vi "TLB Native Dynamic Events ver 0.26e.vi"() -> ()   [LabVIEW 2018] (continued)
                # "Stays in Task 5D until the object is detected"
                # "T: Go back to idle, F: Continue with task\""
                # ">> Manual override >>"
                n445 = case shown="False" w1151 {
                  tunnel: [w1164 w1170] -> w1160
                  tunnel: w1152 -> [w1162 w1168]
                  frame False {
                    n446 = for {
                      tunnel: string[] ["START TIMER", "OPEN CLAW", ""] ("element") -> [w1165] mode=indexing
                      shift-right: [w1167] -> w1164
                      shift-left: w1162 -> [w1166]
                      n447 = Enqueue Element(queue=w1166, element=w1165) -> (queue out=w1167:refnum<queue>)  [unwired: 2 in, 2 out]
                    }
                  }
                  frame True {
                    n448 = for {
                      shift-right: [w1172] -> w1170
                      shift-left: w1168 -> [w1173]
                      tunnel: string[] ["CAM CLOSE", "", ""] -> [w1171] mode=indexing
                      n449 = Enqueue Element(queue=w1173, element=w1171) -> (queue out=w1172:refnum<queue>)  [unwired: 2 in, 2 out]
                    }
                  }
                }
                n450 = Or(x=w1151, y=w1156) -> (x .or. y?=w1158:bool)
                n451 = Select(t=State_Type_Definitions,_for_0.26g_versions_and_later_2."True Stop" ("Enum"), s=w1156, f=State_Type_Definitions,_for_0.26g_versions_and_later_2."True Stop" ("Enum")) -> (s? t:f=w1153:T18)
                n452 = Select(t=w1153, s=w1158, f=State_Type_Definitions,_for_0.26g_versions_and_later_2."Task 5D" ("Enum")) -> (s? t:f=w1157:T18)
              }
              frame "Exit" {
                n453 = for {
                  shift-right: [w1180] -> w1177
                  shift-left: w1174 -> [w1181]
                  tunnel: string[] ["STOP", "RESET ENCODERS", "RESET YAW", "ARDUINO MODE 0"] -> [w1179] mode=indexing
                  n454 = Enqueue Element(queue=w1181, element=w1179) -> (queue out=w1180:refnum<queue>)  [unwired: 2 in, 2 out]
                }
              }
            }
          }
          frame 20 {
            # ">>> yStepper command>>>"
            n455 = Dequeue Element(queue=w1195, timeout in ms (-1)=w1196, error in (no error)=w1197) -> (element=w1199:T10)  [unwired: 3 out]
            n456 = formula code="if (pos < 100)\ny = 41;\n\nelse if (pos >= 100 && pos <= 140)\ny = 30;\n\nelse if (pos >= 141 && pos <= 170)\ny = 25;\n\nelse if (pos >= 171 &&pos <= 180) \ny = 20;\n\nelse if (pos >= 181&& pos <= 200)\ny = 15;\n\nelse if (pos >= 201 && pos <= 230)\ny = 10;\n\nelse if (pos >= 231 && pos <= 320)\ny = 8;\n\nelse if (pos > 320)\ny = 0;"("pos"=w1187) -> ("y"=w1190:dbl)
            n457 = To Unsigned Byte Integer(number=w1190) -> (unsigned 8bit integer=w1185:u8)
            n458 = Equal?(x=w1186, y=w1185) -> (x = y?=w1184:bool)
            n459 = case shown="\"Start Task 1\", Default" w1199 {
              tunnel: [w1206 State_Type_Definitions,_for_0.26g_versions_and_later_2."True Stop" ("Enum")] -> w1193
              tunnel: [w1209 w1226] -> w1191
              tunnel: [State_Type_Definitions,_for_0.26g_versions_and_later_2."Idle" ("Enum") State_Type_Definitions,_for_0.26g_versions_and_later_2."Shutdown" ("Enum")] -> w1192
              tunnel: w1198 -> [w1205 _]
              tunnel: w1194 -> [w1201 w1223]
              tunnel: w1184 -> [w1200 _]
              frame "Start Task 1", Default {
                # ">> T: Breaks out of state loop; F: Stays in loop>>"
                # ">> Manual override >>"
                # ">> Checks if time is up>>"
                # "Stays in Task 5D until the object is detected"
                # "T: Go back to idle, F: Continue with task\""
                # ">> Manual override >>"
                n460 = case shown="False" w1200 {
                  tunnel: [w1213 w1219] -> w1209
                  tunnel: w1201 -> [w1211 w1217]
                  frame False {
                    n461 = for {
                      tunnel: string[] ["READ STEPPER VALUES", "Y STEPPER CONTROL", ""] ("element") -> [w1214] mode=indexing
                      shift-right: [w1216] -> w1213
                      shift-left: w1211 -> [w1215]
                      n462 = Enqueue Element(queue=w1215, element=w1214) -> (queue out=w1216:refnum<queue>)  [unwired: 2 in, 2 out]
                    }
                  }
                  frame True {
                    n463 = for {
                      shift-right: [w1221] -> w1219
                      shift-left: w1217 -> [w1222]
                      tunnel: string[] ["CAM CLOSE", "DISPOSE BUFFERS", ""] -> [w1220] mode=indexing
                      n464 = Enqueue Element(queue=w1222, element=w1220) -> (queue out=w1221:refnum<queue>)  [unwired: 2 in, 2 out]
                    }
                  }
                }
                n465 = Or(x=w1200, y=w1205) -> (x .or. y?=w1207:bool)
                n466 = Select(t=State_Type_Definitions,_for_0.26g_versions_and_later_2."True Stop" ("Enum"), s=w1205, f=State_Type_Definitions,_for_0.26g_versions_and_later_2."Task 5F: ARM GRAB HEIGHT" ("Enum")) -> (s? t:f=w1202:T18)
                n467 = Select(t=w1202, s=w1207, f=State_Type_Definitions,_for_0.26g_versions_and_later_2."Task 5E: POSITION ARM" ("Enum")) -> (s? t:f=w1206:T18)
              }
              frame "Exit" {
                n468 = for {
                  shift-right: [w1229] -> w1226
                  shift-left: w1223 -> [w1230]
                  tunnel: string[] ["STOP", "RESET ENCODERS", "RESET YAW", "ARDUINO MODE 0"] -> [w1228] mode=indexing
                  n469 = Enqueue Element(queue=w1230, element=w1228) -> (queue out=w1229:refnum<queue>)  [unwired: 2 in, 2 out]
                }
              }
            }
            n470 = Bundle By Name(cluster=w1189, "yStepper desired"=w1185) -> (w1188:T20)
          }
          frame 21 {
            # ">>> Motor control cluster >>>"
            # ">>> yStepper command>>>"
            # ">> Manual override >>"
            n471 = Dequeue Element(queue=w1241, timeout in ms (-1)=w1240, error in (no error)=w1242) -> (element=w1239:T10)  [unwired: 3 out]
            n472 = Equal?(x=w1238, y=u8 1) -> (x = y?=w1236:bool)
            n473 = case shown="\"Start Task 1\", Default" w1239 {
              tunnel: [w1252 State_Type_Definitions,_for_0.26g_versions_and_later_2."True Stop" ("Enum")] -> w1243
              tunnel: [w1255 w1272] -> w1244
              tunnel: [State_Type_Definitions,_for_0.26g_versions_and_later_2."Idle" ("Enum") State_Type_Definitions,_for_0.26g_versions_and_later_2."Shutdown" ("Enum")] -> w1245
              tunnel: w1236 -> [w1251 _]
              tunnel: w1235 -> [w1250 _]
              tunnel: w1234 -> [w1246 w1269]
              frame "Start Task 1", Default {
                # "Stays in Task 5F until stepper reaches desired \nheight"
                # "T: Go back to idle, F: Continue with task\""
                # ">> Manual override >>"
                n474 = case shown="True" w1251 {
                  tunnel: [w1259 w1265] -> w1255
                  tunnel: w1246 -> [w1257 w1263]
                  frame False {
                    n475 = for {
                      tunnel: string[] ["Z STEPPER GRAB HEIGHT", "READ STEPPER VALUES"] ("element") -> [w1260] mode=indexing
                      shift-right: [w1262] -> w1259
                      shift-left: w1257 -> [w1261]
                      n476 = Enqueue Element(queue=w1261, element=w1260) -> (queue out=w1262:refnum<queue>)  [unwired: 2 in, 2 out]
                    }
                  }
                  frame True {
                    n477 = for {
                      shift-right: [w1267] -> w1265
                      shift-left: w1263 -> [w1268]
                      tunnel: string[] ["SET TIMER 5", "CLOSE CLAW", ""] -> [w1266] mode=indexing
                      n478 = Enqueue Element(queue=w1268, element=w1266) -> (queue out=w1267:refnum<queue>)  [unwired: 2 in, 2 out]
                    }
                  }
                }
                n479 = Or(x=w1251, y=w1250) -> (x .or. y?=w1253:bool)
                n480 = Select(t=State_Type_Definitions,_for_0.26g_versions_and_later_2."True Stop" ("Enum"), s=w1250, f=State_Type_Definitions,_for_0.26g_versions_and_later_2."Task 5G: CLOSE CLAW" ("Enum")) -> (s? t:f=w1247:T18)
                n481 = Select(t=w1247, s=w1253, f=State_Type_Definitions,_for_0.26g_versions_and_later_2."Task 5F: ARM GRAB HEIGHT" ("Enum")) -> (s? t:f=w1252:T18)
              }
              frame "Exit" {
                n482 = for {
                  shift-right: [w1275] -> w1272
                  shift-left: w1269 -> [w1276]
                  tunnel: string[] ["STOP", "RESET ENCODERS", "RESET YAW", "ARDUINO MODE 0"] -> [w1274] mode=indexing
                  n483 = Enqueue Element(queue=w1276, element=w1274) -> (queue out=w1275:refnum<queue>)  [unwired: 2 in, 2 out]
                }
              }
            }
          }
          frame 22 {
            # ">>> yStepper command>>>"
            # ">> Manual override >>"
            n484 = Dequeue Element(queue=w1287, timeout in ms (-1)=w1286, error in (no error)=w1285) -> (element=w1284:T10)  [unwired: 3 out]
            n485 = case shown="\"Start Task 1\", Default" w1284 {
              tunnel: [w1296 State_Type_Definitions,_for_0.26g_versions_and_later_2."True Stop" ("Enum")] -> w1289
              tunnel: [w1299 w1316] -> w1282
              tunnel: [State_Type_Definitions,_for_0.26g_versions_and_later_2."Idle" ("Enum") State_Type_Definitions,_for_0.26g_versions_and_later_2."Shutdown" ("Enum")] -> w1281
              tunnel: w1283 -> [w1290 _]
              tunnel: w1288 -> [w1295 w1313]
              tunnel: w1279 -> [w1294 _]
              frame "Start Task 1", Default {
                # ">> Is time up? >>"
                # "Determines if object is in range to pick up"
                # ">> Manual override >>"
                n486 = case shown="True" w1294 {
                  tunnel: [w1303 w1309] -> w1299
                  tunnel: w1295 -> [w1301 w1307]
                  frame False {
                    n487 = for {
                      tunnel: string[] ["CLOSE CLAW", "START TIMER"] ("element") -> [w1304] mode=indexing
                      shift-right: [w1306] -> w1303
                      shift-left: w1301 -> [w1305]
                      n488 = Enqueue Element(queue=w1305, element=w1304) -> (queue out=w1306:refnum<queue>)  [unwired: 2 in, 2 out]
                    }
                  }
                  frame True {
                    n489 = for {
                      shift-right: [w1311] -> w1309
                      shift-left: w1307 -> [w1312]
                      tunnel: string[] ["READ STEPPER VALUES", "", ""] -> [w1310] mode=indexing
                      n490 = Enqueue Element(queue=w1312, element=w1310) -> (queue out=w1311:refnum<queue>)  [unwired: 2 in, 2 out]
                    }
                  }
                }
                n491 = Or(x=w1294, y=w1290) -> (x .or. y?=w1297:bool)
                n492 = Select(t=State_Type_Definitions,_for_0.26g_versions_and_later_2."True Stop" ("Enum"), s=w1290, f=State_Type_Definitions,_for_0.26g_versions_and_later_2."Task 5H: RAISE ARM" ("Enum")) -> (s? t:f=w1292:T18)
                n493 = Select(t=w1292, s=w1297, f=State_Type_Definitions,_for_0.26g_versions_and_later_2."Task 5G: CLOSE CLAW" ("Enum")) -> (s? t:f=w1296:T18)
              }
              frame "Exit" {
                n494 = for {
                  shift-right: [w1319] -> w1316
                  shift-left: w1313 -> [w1320]
                  tunnel: string[] ["STOP", "RESET ENCODERS", "RESET YAW", "ARDUINO MODE 0"] -> [w1318] mode=indexing
                  n495 = Enqueue Element(queue=w1320, element=w1318) -> (queue out=w1319:refnum<queue>)  [unwired: 2 in, 2 out]
                }
              }
            }
          }
          frame 23 {
            # ">>> yStepper command>>>"
            # ">> Manual override >>"
            n496 = Dequeue Element(queue=w1331, timeout in ms (-1)=w1330, error in (no error)=w1332) -> (element=w1329:T10)  [unwired: 3 out]
            n497 = Equal?(x=w1328, y=u8 60) -> (x = y?=w1326:bool)
            n498 = case shown="\"Start Task 1\", Default" w1329 {
              tunnel: [w1342 State_Type_Definitions,_for_0.26g_versions_and_later_2."True Stop" ("Enum")] -> w1333
              tunnel: [w1345 w1362] -> w1334
              tunnel: [State_Type_Definitions,_for_0.26g_versions_and_later_2."Idle" ("Enum") State_Type_Definitions,_for_0.26g_versions_and_later_2."Shutdown" ("Enum")] -> w1335
              tunnel: w1326 -> [w1341 _]
              tunnel: w1325 -> [w1340 _]
              tunnel: w1324 -> [w1336 w1359]
              frame "Start Task 1", Default {
                # "Stays in Task 5_A until stepper reaches desired \nheight"
                # "T: Go back to idle, F: Continue with task\""
                # ">> Manual override >>"
                n499 = case shown="False" w1341 {
                  tunnel: [w1349 w1355] -> w1345
                  tunnel: w1336 -> [w1347 w1353]
                  frame False {
                    n500 = for {
                      tunnel: string[] ["Z STEPPER CAM HEIGHT", "READ STEPPER VALUES"] ("element") -> [w1350] mode=indexing
                      shift-right: [w1352] -> w1349
                      shift-left: w1347 -> [w1351]
                      n501 = Enqueue Element(queue=w1351, element=w1350) -> (queue out=w1352:refnum<queue>)  [unwired: 2 in, 2 out]
                    }
                  }
                  frame True {
                    n502 = for {
                      shift-right: [w1357] -> w1355
                      shift-left: w1353 -> [w1358]
                      tunnel: string[] ["ARDUINO - ULTRASONIC", "READ ULTRASONIC", ""] -> [w1356] mode=indexing
                      n503 = Enqueue Element(queue=w1358, element=w1356) -> (queue out=w1357:refnum<queue>)  [unwired: 2 in, 2 out]
                    }
                  }
                }
                n504 = Or(x=w1341, y=w1340) -> (x .or. y?=w1343:bool)
                n505 = Select(t=State_Type_Definitions,_for_0.26g_versions_and_later_2."True Stop" ("Enum"), s=w1340, f=State_Type_Definitions,_for_0.26g_versions_and_later_2."True Stop" ("Enum")) -> (s? t:f=w1337:T18)
                n506 = Select(t=w1337, s=w1343, f=State_Type_Definitions,_for_0.26g_versions_and_later_2."Task 5H: RAISE ARM" ("Enum")) -> (s? t:f=w1342:T18)
              }
              frame "Exit" {
                n507 = for {
                  shift-right: [w1365] -> w1362
                  shift-left: w1359 -> [w1366]
                  tunnel: string[] ["STOP", "RESET ENCODERS", "RESET YAW", "ARDUINO MODE 0"] -> [w1364] mode=indexing
                  n508 = Enqueue Element(queue=w1366, element=w1364) -> (queue out=w1365:refnum<queue>)  [unwired: 2 in, 2 out]
                }
              }
            }
          }
          frame 24 {
            # ">>> yStepper command>>>"
            n509 = Dequeue Element(queue=w1376, timeout in ms (-1)=w1375, error in (no error)=w1374) -> (element=w1381:T10)  [unwired: 3 out]
            n510 = Equal?(x=w1372, y=u8 60) -> (x = y?=w1371:bool)
            n511 = case shown="\"Start Task 1\", Default" w1381 {
              tunnel: [w1388 State_Type_Definitions,_for_0.26g_versions_and_later_2."True Stop" ("Enum")] -> w1379
              tunnel: [w1387 w1405] -> w1378
              tunnel: [State_Type_Definitions,_for_0.26g_versions_and_later_2."Idle" ("Enum") State_Type_Definitions,_for_0.26g_versions_and_later_2."Shutdown" ("Enum")] -> w1380
              tunnel: w1377 -> [w1383 _]
              tunnel: w1373 -> [w1385 _]
              tunnel: w1371 -> [w1382 _]
              frame "Start Task 1", Default {
                n512 = case shown="False" w1382 {
                  tunnel: [w1393 w1399] -> w1387
                  tunnel: w1385 -> [w1391 w1397]
                  frame False {
                    n513 = for {
                      tunnel: string[] ["Z STEPPER CAM HEIGHT", "READ STEPPER VALUES"] ("element") -> [w1394] mode=indexing
                      shift-right: [w1396] -> w1393
                      shift-left: w1391 -> [w1395]
                      n514 = Enqueue Element(queue=w1395, element=w1394) -> (queue out=w1396:refnum<queue>)  [unwired: 2 in, 2 out]
                    }
                  }
                  frame True {
                    n515 = for {
                      shift-right: [w1401] -> w1399
                      shift-left: w1397 -> [w1402]
                      tunnel: string[] ["CAM ACQ", "OPEN LOG CAM"] -> [w1400] mode=indexing
                      n516 = Enqueue Element(queue=w1402, element=w1400) -> (queue out=w1401:refnum<queue>)  [unwired: 2 in, 2 out]
                    }
                  }
                }
                n517 = Or(x=w1382, y=w1383) -> (x .or. y?=w1384:bool)
                n518 = Select(t=State_Type_Definitions,_for_0.26g_versions_and_later_2."Task 6_B" ("Enum"), s=w1384, f=State_Type_Definitions,_for_0.26g_versions_and_later_2."Task 6_A" ("Enum")) -> (s? t:f=w1388:T18)
              }
              frame "Exit" {
                n519 = for {
                  shift-right: [w1408] -> w1405
                  shift-left: _ -> [w1409]
                  tunnel: string[] ["STOP", "RESET ENCODERS", "RESET YAW", "ARDUINO MODE 0"] -> [w1407] mode=indexing
                  n520 = Enqueue Element(queue=w1409, element=w1407) -> (queue out=w1408:refnum<queue>)  [unwired: 2 in, 2 out]
                }
              }
            }
          }
          frame 25 {
            # ">>> yStepper command>>>"
            n521 = Dequeue Element(queue=w1421, timeout in ms (-1)=w1419, error in (no error)=w1420) -> (element=w1418:T10)  [unwired: 3 out]
            n522 = case shown="\"Start Task 1\", Default" w1418 {
              tunnel: [w1428 State_Type_Definitions,_for_0.26g_versions_and_later_2."True Stop" ("Enum")] -> w1414
              tunnel: [w1427 w1446] -> w1422
              tunnel: [State_Type_Definitions,_for_0.26g_versions_and_later_2."Idle" ("Enum") State_Type_Definitions,_for_0.26g_versions_and_later_2."Shutdown" ("Enum")] -> w1415
              tunnel: w1417 -> [w1423 _]
              tunnel: w1416 -> [w1425 _]
              tunnel: w1413 -> [w1424 w1443]
              frame "Start Task 1", Default {
                # ">> Manual override >>"
                n523 = case shown="False" w1425 {
                  tunnel: [w1433 w1439] -> w1427
                  tunnel: w1424 -> [w1432 w1437]
                  frame False {
                    n524 = for {
                      shift-right: [w1436] -> w1433
                      shift-left: w1432 -> [w1435]
                      tunnel: string[] ["CAM ACQ", "PROCESS IMAGE", "OPEN CLAW"] -> [w1434] mode=indexing
                      n525 = Enqueue Element(queue=w1435, element=w1434) -> (queue out=w1436:refnum<queue>)  [unwired: 2 in, 2 out]
                    }
                  }
                  frame True {
                    n526 = for {
                      shift-right: [w1441] -> w1439
                      shift-left: w1437 -> [w1442]
                      tunnel: string[] ["CAM ACQ", "PROCESS IMAGE", "CLOSE CLAW"] -> [w1440] mode=indexing
                      n527 = Enqueue Element(queue=w1442, element=w1440) -> (queue out=w1441:refnum<queue>)  [unwired: 2 in, 2 out]
                    }
                  }
                }
                n528 = Select(t=State_Type_Definitions,_for_0.26g_versions_and_later_2."True Stop" ("Enum"), s=w1423, f=State_Type_Definitions,_for_0.26g_versions_and_later_2."Task 6_B" ("Enum")) -> (s? t:f=w1428:T18)
              }
              frame "Exit" {
                # ">> State after true stop >>"
                # ">> Goes to true stop >>"
                n529 = for {
                  shift-right: [w1449] -> w1446
                  shift-left: w1443 -> [w1450]
                  tunnel: string[] ["STOP", "RESET ENCODERS", "RESET YAW", ""] -> [w1448] mode=indexing
                  n530 = Enqueue Element(queue=w1450, element=w1448) -> (queue out=w1449:refnum<queue>)  [unwired: 2 in, 2 out]
                }
              }
            }
          }
          frame 26 {
          }
          frame 27 {
            # ">>> Motor control cluster >>>"
            # ">>> yStepper command>>>"
            # ">> Manual override >>"
            n531 = Dequeue Element(queue=w1467, timeout in ms (-1)=w1466, error in (no error)=w1468) -> (element=w1465:T10)  [unwired: 3 out]
            n532 = Equal?(x=w1464, y=u8 60) -> (x = y?=w1462:bool)
            n533 = case shown="\"Start Task 1\", Default" w1465 {
              tunnel: [w1478 State_Type_Definitions,_for_0.26g_versions_and_later_2."True Stop" ("Enum")] -> w1469
              tunnel: [w1481 w1498] -> w1470
              tunnel: [State_Type_Definitions,_for_0.26g_versions_and_later_2."Idle" ("Enum") State_Type_Definitions,_for_0.26g_versions_and_later_2."Shutdown" ("Enum")] -> w1471
              tunnel: w1462 -> [w1477 _]
              tunnel: w1461 -> [w1476 _]
              tunnel: w1460 -> [w1472 w1495]
              frame "Start Task 1", Default {
                # "Stays in Task 5_A until stepper reaches desired \nheight"
                # "T: Go back to idle, F: Continue with task\""
                # ">> Manual override >>"
                n534 = case shown="True" w1477 {
                  tunnel: [w1485 w1491] -> w1481
                  tunnel: w1472 -> [w1483 w1489]
                  frame False {
                    n535 = for {
                      tunnel: string[] ["Z STEPPER CAM HEIGHT", "READ STEPPER VALUES"] ("element") -> [w1486] mode=indexing
                      shift-right: [w1488] -> w1485
                      shift-left: w1483 -> [w1487]
                      n536 = Enqueue Element(queue=w1487, element=w1486) -> (queue out=w1488:refnum<queue>)  [unwired: 2 in, 2 out]
                    }
                  }
                  frame True {
                    n537 = for {
                      shift-right: [w1493] -> w1491
                      shift-left: w1489 -> [w1494]
                      tunnel: string[] ["RESET YAW", "RESET ENCODERS", "READ IR"] -> [w1492] mode=indexing
                      n538 = Enqueue Element(queue=w1494, element=w1492) -> (queue out=w1493:refnum<queue>)  [unwired: 2 in, 2 out]
                    }
                  }
                }
                n539 = Or(x=w1477, y=w1476) -> (x .or. y?=w1479:bool)
                n540 = Select(t=State_Type_Definitions,_for_0.26g_versions_and_later_2."True Stop" ("Enum"), s=w1476, f=State_Type_Definitions,_for_0.26g_versions_and_later_2."Task 8B: MOVE TO BOX" ("Enum")) -> (s? t:f=w1473:T18)
                n541 = Select(t=w1473, s=w1479, f=State_Type_Definitions,_for_0.26g_versions_and_later_2."Task 8A: RAISE ARM" ("Enum")) -> (s? t:f=w1478:T18)
              }
              frame "Exit" {
                n542 = for {
                  shift-right: [w1501] -> w1498
                  shift-left: w1495 -> [w1502]
                  tunnel: string[] ["STOP", "RESET ENCODERS", "RESET YAW", "ARDUINO MODE 0"] -> [w1500] mode=indexing
                  n543 = Enqueue Element(queue=w1502, element=w1500) -> (queue out=w1501:refnum<queue>)  [unwired: 2 in, 2 out]
                }
              }
            }
          }
          frame 28 {
            w1512 = u8 15 ("y")
            # ">>> yStepper command>>>"
            n544 = Less?(x=w1509, y=w1512) -> (x < y?=w1510:bool)
            n545 = Dequeue Element(queue=w1516, timeout in ms (-1)=w1515, error in (no error)=w1517) -> (element=w1514:T10)  [unwired: 3 out]
            n546 = Less?(x=w1508, y=w1512) -> (x < y?=w1511:bool)
            n547 = Less?(x=w1505, y=50.0) -> (x < y?=w1503:bool)
            n548 = And(x=w1511, y=w1510) -> ()  [unwired: 1 out]
            n549 = case shown="\"Start Task 1\", Default" w1514 {
              tunnel: [w1529 State_Type_Definitions,_for_0.26g_versions_and_later_2."True Stop" ("Enum")] -> w1519
              tunnel: [w1532 w1549] -> w1518
              tunnel: [State_Type_Definitions,_for_0.26g_versions_and_later_2."Idle" ("Enum") State_Type_Definitions,_for_0.26g_versions_and_later_2."Shutdown" ("Enum")] -> w1520
              tunnel: w1522 -> [w1528 _]
              tunnel: w1521 -> [w1524 w1546]
              tunnel: w1503 -> [w1523 _]
              frame "Start Task 1", Default {
                # "Stays in Task 5_B to capture image over 5 seconds"
                # "T: Go back to idle, F: Continue with task\""
                # ">> Manual override >>"
                n550 = case shown="True" w1523 {
                  tunnel: [w1536 w1542] -> w1532
                  tunnel: w1524 -> [w1534 w1540]
                  frame False {
                    n551 = for {
                      tunnel: string[] ["FORWARD", "READ IR", "READ NAVX"] ("element") -> [w1537] mode=indexing
                      shift-right: [w1539] -> w1536
                      shift-left: w1534 -> [w1538]
                      n552 = Enqueue Element(queue=w1538, element=w1537) -> (queue out=w1539:refnum<queue>)  [unwired: 2 in, 2 out]
                    }
                  }
                  frame True {
                    n553 = for {
                      shift-right: [w1544] -> w1542
                      shift-left: w1540 -> [w1545]
                      tunnel: string[] ["STOP", "RESET ENCODERS", "OPEN LOG CAM", "SET TIMER 2", "OPEN IMAQ REF"] -> [w1543] mode=indexing
                      n554 = Enqueue Element(queue=w1545, element=w1543) -> (queue out=w1544:refnum<queue>)  [unwired: 2 in, 2 out]
                    }
                  }
                }
                n555 = Or(x=w1523, y=w1528) -> (x .or. y?=w1530:bool)
                n556 = Select(t=State_Type_Definitions,_for_0.26g_versions_and_later_2."True Stop" ("Enum"), s=w1528, f=State_Type_Definitions,_for_0.26g_versions_and_later_2."Task 8C: CAM BURST" ("Enum")) -> (s? t:f=w1525:T18)
                n557 = Select(t=w1525, s=w1530, f=State_Type_Definitions,_for_0.26g_versions_and_later_2."Task 8B: MOVE TO BOX" ("Enum")) -> (s? t:f=w1529:T18)
              }
              frame "Exit" {
                n558 = for {
                  shift-right: [w1552] -> w1549
                  shift-left: w1546 -> [w1553]
                  tunnel: string[] ["STOP", "RESET ENCODERS", "RESET YAW", "ARDUINO MODE 0"] -> [w1551] mode=indexing
                  n559 = Enqueue Element(queue=w1553, element=w1551) -> (queue out=w1552:refnum<queue>)  [unwired: 2 in, 2 out]
                }
              }
            }
          }
          frame 29 {
            # ">>> Motor control cluster >>>"
            # ">>> yStepper command>>>"
            # ">> Manual override >>"
            n560 = Dequeue Element(queue=w1564, timeout in ms (-1)=w1563, error in (no error)=w1562) -> (element=w1561:T10)  [unwired: 3 out]
            n561 = case shown="\"Start Task 1\", Default" w1561 {
              tunnel: [w1573 State_Type_Definitions,_for_0.26g_versions_and_later_2."True Stop" ("Enum")] -> w1566
              tunnel: [w1576 w1593] -> w1559
              tunnel: [State_Type_Definitions,_for_0.26g_versions_and_later_2."Idle" ("Enum") State_Type_Definitions,_for_0.26g_versions_and_later_2."Shutdown" ("Enum")] -> w1558
              tunnel: w1560 -> [w1567 _]
              tunnel: w1565 -> [w1572 w1590]
              tunnel: w1556 -> [w1571 _]
              frame "Start Task 1", Default {
                # ">> Is time up? >>"
                # "Determines if object is in range to pick up"
                # ">> Manual override >>"
                n562 = case shown="True" w1571 {
                  tunnel: [w1580 w1586] -> w1576
                  tunnel: w1572 -> [w1578 w1584]
                  frame False {
                    n563 = for {
                      tunnel: string[] ["CAM ACQ", "START TIMER"] ("element") -> [w1581] mode=indexing
                      shift-right: [w1583] -> w1580
                      shift-left: w1578 -> [w1582]
                      n564 = Enqueue Element(queue=w1582, element=w1581) -> (queue out=w1583:refnum<queue>)  [unwired: 2 in, 2 out]
                    }
                  }
                  frame True {
                    n565 = for {
                      shift-right: [w1588] -> w1586
                      shift-left: w1584 -> [w1589]
                      tunnel: string[] ["CAM CLOSE", "PROCESS IMAGE", "SET TIMER 2"] -> [w1587] mode=indexing
                      n566 = Enqueue Element(queue=w1589, element=w1587) -> (queue out=w1588:refnum<queue>)  [unwired: 2 in, 2 out]
                    }
                  }
                }
                n567 = Or(x=w1571, y=w1567) -> (x .or. y?=w1574:bool)
                n568 = Select(t=State_Type_Definitions,_for_0.26g_versions_and_later_2."True Stop" ("Enum"), s=w1567, f=State_Type_Definitions,_for_0.26g_versions_and_later_2."Task 8D: PROCESS IMAGE" ("Enum")) -> (s? t:f=w1569:T18)
                n569 = Select(t=w1569, s=w1574, f=State_Type_Definitions,_for_0.26g_versions_and_later_2."Task 8C: CAM BURST" ("Enum")) -> (s? t:f=w1573:T18)
              }
              frame "Exit" {
                n570 = for {
                  shift-right: [w1596] -> w1593
                  shift-left: w1590 -> [w1597]
                  tunnel: string[] ["STOP", "RESET ENCODERS", "RESET YAW", "ARDUINO MODE 0"] -> [w1595] mode=indexing
                  n571 = Enqueue Element(queue=w1597, element=w1595) -> (queue out=w1596:refnum<queue>)  [unwired: 2 in, 2 out]
                }
              }
            }
          }
          frame 30 {
            # ">>> yStepper command>>>"
            n572 = Dequeue Element(queue=w1605, timeout in ms (-1)=w1604, error in (no error)=w1603) -> (element=w1602:T10)  [unwired: 3 out]
            n573 = case shown="\"Start Task 1\", Default" w1602 {
              tunnel: [w1617 State_Type_Definitions,_for_0.26g_versions_and_later_2."True Stop" ("Enum")] -> w1609
              tunnel: [w1620 w1637] -> w1608
              tunnel: [State_Type_Definitions,_for_0.26g_versions_and_later_2."Idle" ("Enum") State_Type_Definitions,_for_0.26g_versions_and_later_2."Shutdown" ("Enum")] -> w1610
              tunnel: w1606 -> [w1616 _]
              tunnel: w1607 -> [w1612 w1634]
              tunnel: w1600 -> [w1611 _]
              frame "Start Task 1", Default {
                # ">> T: Breaks out of state loop; F: Stays in loop>>"
                # ">> Manual override >>"
                # ">> Checks if time is up>>"
                # "Stays in Task 5D until the object is detected"
                # "T: Go back to idle, F: Continue with task\""
                # ">> Manual override >>"
                n574 = case shown="False" w1611 {
                  tunnel: [w1624 w1630] -> w1620
                  tunnel: w1612 -> [w1622 w1628]
                  frame False {
                    n575 = for {
                      tunnel: string[] ["START TIMER", "PROCESS IMAGE", ""] ("element") -> [w1625] mode=indexing
                      shift-right: [w1627] -> w1624
                      shift-left: w1622 -> [w1626]
                      n576 = Enqueue Element(queue=w1626, element=w1625) -> (queue out=w1627:refnum<queue>)  [unwired: 2 in, 2 out]
                    }
                  }
                  frame True {
                    n577 = for {
                      shift-right: [w1632] -> w1630
                      shift-left: w1628 -> [w1633]
                      tunnel: string[] ["RESET ENCODERS", "", ""] -> [w1631] mode=indexing
                      n578 = Enqueue Element(queue=w1633, element=w1631) -> (queue out=w1632:refnum<queue>)  [unwired: 2 in, 2 out]
                    }
                  }
                }
                n579 = Or(x=w1611, y=w1616) -> (x .or. y?=w1618:bool)
                n580 = Select(t=State_Type_Definitions,_for_0.26g_versions_and_later_2."True Stop" ("Enum"), s=w1616, f=State_Type_Definitions,_for_0.26g_versions_and_later_2."Task 8E: ROBOT ADJUST" ("Enum")) -> (s? t:f=w1613:T18)
                n581 = Select(t=w1613, s=w1618, f=State_Type_Definitions,_for_0.26g_versions_and_later_2."Task 8D: PROCESS IMAGE" ("Enum")) -> (s? t:f=w1617:T18)
              }
              frame "Exit" {
                n582 = for {
                  shift-right: [w1640] -> w1637
                  shift-left: w1634 -> [w1641]
                  tunnel: string[] ["STOP", "RESET ENCODERS", "RESET YAW", "ARDUINO MODE 0"] -> [w1639] mode=indexing
                  n583 = Enqueue Element(queue=w1641, element=w1639) -> (queue out=w1640:refnum<queue>)  [unwired: 2 in, 2 out]
                }
              }
            }
          }
          frame 31 {
            # ">>> Motor control cluster >>>"
            # ">>> yStepper command>>>"
            n584 = Dequeue Element(queue=w1658, timeout in ms (-1)=w1657, error in (no error)=w1656) -> (element=w1655:T10)  [unwired: 3 out]
            n585 = Subtract(x=w1653, y=300.0) -> (x-y=w1651:dbl)
            n586 = formula code="if (error <= -61&&error > -300){\ndistance = -15;\nxSpeed = -30;\n}\n\nelse if (error <= -51 && error >= -60){\ndistance = -10;\nxSpeed = -30;\n}\n\nelse if (error >= -50 && error <= 50){\ndistance = 0;\nxSpeed = 0;\n}\n\nelse if (error >= 51 && error <= 80){\ndistance = 10;\nxSpeed = 30;\n}\n\nelse if (error >= 81 && error <= 100){\ndistance = 15;\nxSpeed = 30;\n}\n\nelse if (error >= 101 && error <= 120){\ndistance = 20;\nxSpeed = 30;\n}\n\nelse if (error >= 121 && error < 300){\ndistance = 25;\nxSpeed = 30;\n}\n\nelse{\ndistance = 0;\nxSpeed = 0;\n}"("error"=w1651) -> ("distance"=w1646:dbl, "xSpeed"=w1648:dbl)
            n587 = formula code="if (target > 0){\nif (current  >= target)\noutput = 1;\n\nelse if (current != target)\noutput = 0;\n}\n\nelse if (target == 0){\nif (current == target)\noutput = 1;\n\nelse if (current != target)\noutput = 0;\n}\n\nelse if (target < 0){\nif (current <= target)\noutput = 1;\n\nelse if (current != target)\noutput = 0;\n}\n\nelse if (current != target)\noutput = 0;"("target"=w1646, "current"=w1647) -> ("output"=w1645:dbl)
            n588 = Bundle By Name(cluster=w1650, "xSpeed"=w1648) -> (w1649:T19)
            n589 = Equal?(x=w1645, y=1.0) -> (x = y?=w1643:bool)
            n590 = case shown="\"Start Task 1\", Default" w1655 {
              tunnel: [w1670 State_Type_Definitions,_for_0.26g_versions_and_later_2."True Stop" ("Enum")] -> w1662
              tunnel: [w1673 w1690] -> w1661
              tunnel: [State_Type_Definitions,_for_0.26g_versions_and_later_2."Idle" ("Enum") State_Type_Definitions,_for_0.26g_versions_and_later_2."Shutdown" ("Enum")] -> w1663
              tunnel: w1659 -> [w1669 _]
              tunnel: w1660 -> [w1665 w1687]
              tunnel: w1643 -> [w1664 _]
              frame "Start Task 1", Default {
                # ">> T: Breaks out of state loop; F: Stays in loop>>"
                # ">> Manual override >>"
                # ">> Checks if time is up>>"
                # "Stays in Task 5D until the object is detected"
                # "T: Go back to idle, F: Continue with task\""
                # ">> Manual override >>"
                n591 = case shown="True" w1664 {
                  tunnel: [w1677 w1683] -> w1673
                  tunnel: w1665 -> [w1675 w1681]
                  frame False {
                    n592 = for {
                      tunnel: string[] ["X AXIS - SLOW", "READ ENCODERS", "READ NAVX"] ("element") -> [w1678] mode=indexing
                      shift-right: [w1680] -> w1677
                      shift-left: w1675 -> [w1679]
                      n593 = Enqueue Element(queue=w1679, element=w1678) -> (queue out=w1680:refnum<queue>)  [unwired: 2 in, 2 out]
                    }
                  }
                  frame True {
                    n594 = for {
                      shift-right: [w1685] -> w1683
                      shift-left: w1681 -> [w1686]
                      tunnel: string[] ["SET TIMER 2", "STOP", "READ STEPPER VALUES", ""] -> [w1684] mode=indexing
                      n595 = Enqueue Element(queue=w1686, element=w1684) -> (queue out=w1685:refnum<queue>)  [unwired: 2 in, 2 out]
                    }
                  }
                }
                n596 = Or(x=w1664, y=w1669) -> (x .or. y?=w1671:bool)
                n597 = Select(t=State_Type_Definitions,_for_0.26g_versions_and_later_2."True Stop" ("Enum"), s=w1669, f=State_Type_Definitions,_for_0.26g_versions_and_later_2."Task 8H: ARM ADJUST" ("Enum")) -> (s? t:f=w1666:T18)
                n598 = Select(t=w1666, s=w1671, f=State_Type_Definitions,_for_0.26g_versions_and_later_2."Task 8E: ROBOT ADJUST" ("Enum")) -> (s? t:f=w1670:T18)
              }
              frame "Exit" {
                n599 = for {
                  shift-right: [w1693] -> w1690
                  shift-left: w1687 -> [w1694]
                  tunnel: string[] ["STOP", "RESET ENCODERS", "RESET YAW", "ARDUINO MODE 0"] -> [w1692] mode=indexing
                  n600 = Enqueue Element(queue=w1694, element=w1692) -> (queue out=w1693:refnum<queue>)  [unwired: 2 in, 2 out]
                }
              }
            }
          }
          frame 32 {
            # ">>> Motor control cluster >>>"
            # ">>> yStepper command>>>"
            # ">> Manual override >>"
            n601 = Dequeue Element(queue=w1705, timeout in ms (-1)=w1704, error in (no error)=w1703) -> (element=w1702:T10)  [unwired: 3 out]
            n602 = case shown="\"Start Task 1\", Default" w1702 {
              tunnel: [w1714 State_Type_Definitions,_for_0.26g_versions_and_later_2."True Stop" ("Enum")] -> w1707
              tunnel: [w1717 w1734] -> w1700
              tunnel: [State_Type_Definitions,_for_0.26g_versions_and_later_2."Idle" ("Enum") State_Type_Definitions,_for_0.26g_versions_and_later_2."Shutdown" ("Enum")] -> w1699
              tunnel: w1701 -> [w1708 _]
              tunnel: w1706 -> [w1713 w1731]
              tunnel: w1697 -> [w1712 _]
              frame "Start Task 1", Default {
                # ">> Is time up? >>"
                # "Determines if object is in range to pick up"
                # ">> Manual override >>"
                n603 = case shown="False" w1712 {
                  tunnel: [w1721 w1727] -> w1717
                  tunnel: w1713 -> [w1719 w1725]
                  frame False {
                    n604 = for {
                      tunnel: string[] ["CAM ACQ", "START TIMER"] ("element") -> [w1722] mode=indexing
                      shift-right: [w1724] -> w1721
                      shift-left: w1719 -> [w1723]
                      n605 = Enqueue Element(queue=w1723, element=w1722) -> (queue out=w1724:refnum<queue>)  [unwired: 2 in, 2 out]
                    }
                  }
                  frame True {
                    n606 = for {
                      shift-right: [w1729] -> w1727
                      shift-left: w1725 -> [w1730]
                      tunnel: string[] ["CAM CLOSE", "PROCESS IMAGE", "SET TIMER 3"] -> [w1728] mode=indexing
                      n607 = Enqueue Element(queue=w1730, element=w1728) -> (queue out=w1729:refnum<queue>)  [unwired: 2 in, 2 out]
                    }
                  }
                }
                n608 = Or(x=w1712, y=w1708) -> (x .or. y?=w1715:bool)
                n609 = Select(t=State_Type_Definitions,_for_0.26g_versions_and_later_2."True Stop" ("Enum"), s=w1708, f=State_Type_Definitions,_for_0.26g_versions_and_later_2."Task 8G: PROCESS IMAGE 2" ("Enum")) -> (s? t:f=w1710:T18)
                n610 = Select(t=w1710, s=w1715, f=State_Type_Definitions,_for_0.26g_versions_and_later_2."Task 8F: CAM BURST 2" ("Enum")) -> (s? t:f=w1714:T18)
              }
              frame "Exit" {
                n611 = for {
                  shift-right: [w1737] -> w1734
                  shift-left: w1731 -> [w1738]
                  tunnel: string[] ["STOP", "RESET ENCODERS", "RESET YAW", "ARDUINO MODE 0"] -> [w1736] mode=indexing
                  n612 = Enqueue Element(queue=w1738, element=w1736) -> (queue out=w1737:refnum<queue>)  [unwired: 2 in, 2 out]
                }
              }
            }
          }
          frame 33 {
            # ">>> yStepper command>>>"
            n613 = Dequeue Element(queue=w1746, timeout in ms (-1)=w1745, error in (no error)=w1744) -> (element=w1743:T10)  [unwired: 3 out]
            n614 = case shown="\"Start Task 1\", Default" w1743 {
              tunnel: [w1758 State_Type_Definitions,_for_0.26g_versions_and_later_2."True Stop" ("Enum")] -> w1750
              tunnel: [w1761 w1778] -> w1749
              tunnel: [State_Type_Definitions,_for_0.26g_versions_and_later_2."Idle" ("Enum") State_Type_Definitions,_for_0.26g_versions_and_later_2."Shutdown" ("Enum")] -> w1751
              tunnel: w1747 -> [w1757 _]
              tunnel: w1748 -> [w1753 w1775]
              tunnel: w1741 -> [w1752 _]
              frame "Start Task 1", Default {
                # ">> T: Breaks out of state loop; F: Stays in loop>>"
                # ">> Manual override >>"
                # ">> Checks if time is up>>"
                # "Stays in Task 5D until the object is detected"
                # "T: Go back to idle, F: Continue with task\""
                # ">> Manual override >>"
                n615 = case shown="False" w1752 {
                  tunnel: [w1765 w1771] -> w1761
                  tunnel: w1753 -> [w1763 w1769]
                  frame False {
                    n616 = for {
                      tunnel: string[] ["START TIMER", "PROCESS IMAGE", ""] ("element") -> [w1766] mode=indexing
                      shift-right: [w1768] -> w1765
                      shift-left: w1763 -> [w1767]
                      n617 = Enqueue Element(queue=w1767, element=w1766) -> (queue out=w1768:refnum<queue>)  [unwired: 2 in, 2 out]
                    }
                  }
                  frame True {
                    n618 = for {
                      shift-right: [w1773] -> w1771
                      shift-left: w1769 -> [w1774]
                      tunnel: string[] ["READ STEPPER VALUES", "Y STEPPER CONTROL", ""] -> [w1772] mode=indexing
                      n619 = Enqueue Element(queue=w1774, element=w1772) -> (queue out=w1773:refnum<queue>)  [unwired: 2 in, 2 out]
                    }
                  }
                }
                n620 = Or(x=w1752, y=w1757) -> (x .or. y?=w1759:bool)
                n621 = Select(t=State_Type_Definitions,_for_0.26g_versions_and_later_2."True Stop" ("Enum"), s=w1757, f=State_Type_Definitions,_for_0.26g_versions_and_later_2."Task 8H: ARM ADJUST" ("Enum")) -> (s? t:f=w1754:T18)
                n622 = Select(t=w1754, s=w1759, f=State_Type_Definitions,_for_0.26g_versions_and_later_2."Task 8G: PROCESS IMAGE 2" ("Enum")) -> (s? t:f=w1758:T18)
              }
              frame "Exit" {
                n623 = for {
                  shift-right: [w1781] -> w1778
                  shift-left: w1775 -> [w1782]
                  tunnel: string[] ["STOP", "RESET ENCODERS", "RESET YAW", "ARDUINO MODE 0"] -> [w1780] mode=indexing
                  n624 = Enqueue Element(queue=w1782, element=w1780) -> (queue out=w1781:refnum<queue>)  [unwired: 2 in, 2 out]
                }
              }
            }
          }
          frame 34 {
            # ">>> yStepper command>>>"
            n625 = Dequeue Element(queue=w1796, timeout in ms (-1)=w1797, error in (no error)=w1798) -> (element=w1800:T10)  [unwired: 3 out]
            n626 = formula code="if (pos < 70)\ny = 43;\n\nelse if (pos >= 71 &&pos <= 80)\ny = 40;\n\nelse if (pos >= 81 && pos <= 90)\ny = 38;\n\nelse if (pos >= 91 &&pos <= 120)\ny = 35;\n\nelse if (pos >= 121 && pos <= 140)\ny = 30;\n\nelse if (pos >= 141 && pos <= 170)\ny = 26;\n\nelse if (pos >= 171 &&pos <= 220) \ny = 20;\n\nelse if (pos >= 221&& pos <= 240)\ny = 15;\n\nelse if (pos >= 241 && pos <= 250)\ny = 10;\n\nelse if (pos >= 251)\ny = 0;"("pos"=w1788) -> ("y"=w1791:dbl)
            n627 = To Unsigned Byte Integer(number=w1791) -> (unsigned 8bit integer=w1786:u8)
            n628 = Equal?(x=w1787, y=w1786) -> (x = y?=w1785:bool)
            n629 = case shown="\"Start Task 1\", Default" w1800 {
              tunnel: [w1807 State_Type_Definitions,_for_0.26g_versions_and_later_2."True Stop" ("Enum")] -> w1794
              tunnel: [w1810 w1827] -> w1792
              tunnel: [State_Type_Definitions,_for_0.26g_versions_and_later_2."Idle" ("Enum") State_Type_Definitions,_for_0.26g_versions_and_later_2."Shutdown" ("Enum")] -> w1793
              tunnel: w1799 -> [w1806 _]
              tunnel: w1795 -> [w1802 w1824]
              tunnel: w1785 -> [w1801 _]
              frame "Start Task 1", Default {
                # ">> T: Breaks out of state loop; F: Stays in loop>>"
                # ">> Manual override >>"
                # ">> Checks if time is up>>"
                # "Stays in Task 5D until the object is detected"
                # "T: Go back to idle, F: Continue with task\""
                # ">> Manual override >>"
                n630 = case shown="False" w1801 {
                  tunnel: [w1814 w1820] -> w1810
                  tunnel: w1802 -> [w1812 w1818]
                  frame False {
                    n631 = for {
                      tunnel: string[] ["READ STEPPER VALUES", "Y STEPPER CONTROL", ""] ("element") -> [w1815] mode=indexing
                      shift-right: [w1817] -> w1814
                      shift-left: w1812 -> [w1816]
                      n632 = Enqueue Element(queue=w1816, element=w1815) -> (queue out=w1817:refnum<queue>)  [unwired: 2 in, 2 out]
                    }
                  }
                  frame True {
                    n633 = for {
                      shift-right: [w1822] -> w1820
                      shift-left: w1818 -> [w1823]
                      tunnel: string[] ["DISPOSE BUFFERS", "READ STEPPER VALUES", ""] -> [w1821] mode=indexing
                      n634 = Enqueue Element(queue=w1823, element=w1821) -> (queue out=w1822:refnum<queue>)  [unwired: 2 in, 2 out]
                    }
                  }
                }
                n635 = Or(x=w1801, y=w1806) -> (x .or. y?=w1808:bool)
                n636 = Select(t=State_Type_Definitions,_for_0.26g_versions_and_later_2."True Stop" ("Enum"), s=w1806, f=State_Type_Definitions,_for_0.26g_versions_and_later_2."Task 8I: ARM GRAB HEIGHT" ("Enum")) -> (s? t:f=w1803:T18)
                n637 = Select(t=w1803, s=w1808, f=State_Type_Definitions,_for_0.26g_versions_and_later_2."Task 8H: ARM ADJUST" ("Enum")) -> (s? t:f=w1807:T18)
              }
              frame "Exit" {
                n638 = for {
                  shift-right: [w1830] -> w1827
                  shift-left: w1824 -> [w1831]
                  tunnel: string[] ["STOP", "RESET ENCODERS", "RESET YAW", "ARDUINO MODE 0"] -> [w1829] mode=indexing
                  n639 = Enqueue Element(queue=w1831, element=w1829) -> (queue out=w1830:refnum<queue>)  [unwired: 2 in, 2 out]
                }
              }
            }
            n640 = Bundle By Name(cluster=w1790, "yStepper desired"=w1786) -> (w1789:T20)
          }
          frame 35 {
            # ">>> Motor control cluster >>>"
            # ">>> yStepper command>>>"
            # ">> Manual override >>"
            n641 = Dequeue Element(queue=w1842, timeout in ms (-1)=w1841, error in (no error)=w1843) -> (element=w1840:T10)  [unwired: 3 out]
            n642 = Equal?(x=w1839, y=u8 1) -> (x = y?=w1837:bool)
            n643 = case shown="\"Start Task 1\", Default" w1840 {
              tunnel: [w1853 State_Type_Definitions,_for_0.26g_versions_and_later_2."True Stop" ("Enum")] -> w1844
              tunnel: [w1856 w1873] -> w1845
              tunnel: [State_Type_Definitions,_for_0.26g_versions_and_later_2."Idle" ("Enum") State_Type_Definitions,_for_0.26g_versions_and_later_2."Shutdown" ("Enum")] -> w1846
              tunnel: w1837 -> [w1852 _]
              tunnel: w1836 -> [w1851 _]
              tunnel: w1835 -> [w1847 w1870]
              frame "Start Task 1", Default {
                # "Stays in Task 5F until stepper reaches desired \nheight"
                # "T: Go back to idle, F: Continue with task\""
                # ">> Manual override >>"
                n644 = case shown="True" w1852 {
                  tunnel: [w1860 w1866] -> w1856
                  tunnel: w1847 -> [w1858 w1864]
                  frame False {
                    n645 = for {
                      tunnel: string[] ["Z STEPPER GRAB HEIGHT", "READ STEPPER VALUES"] ("element") -> [w1861] mode=indexing
                      shift-right: [w1863] -> w1860
                      shift-left: w1858 -> [w1862]
                      n646 = Enqueue Element(queue=w1862, element=w1861) -> (queue out=w1863:refnum<queue>)  [unwired: 2 in, 2 out]
                    }
                  }
                  frame True {
                    n647 = for {
                      shift-right: [w1868] -> w1866
                      shift-left: w1864 -> [w1869]
                      tunnel: string[] ["SET TIMER 2", "CLOSE CLAW", ""] -> [w1867] mode=indexing
                      n648 = Enqueue Element(queue=w1869, element=w1867) -> (queue out=w1868:refnum<queue>)  [unwired: 2 in, 2 out]
                    }
                  }
                }
                n649 = Or(x=w1852, y=w1851) -> (x .or. y?=w1854:bool)
                n650 = Select(t=State_Type_Definitions,_for_0.26g_versions_and_later_2."True Stop" ("Enum"), s=w1851, f=State_Type_Definitions,_for_0.26g_versions_and_later_2."Task 8J: CLOSE CLAW" ("Enum")) -> (s? t:f=w1848:T18)
                n651 = Select(t=w1848, s=w1854, f=State_Type_Definitions,_for_0.26g_versions_and_later_2."Task 8I: ARM GRAB HEIGHT" ("Enum")) -> (s? t:f=w1853:T18)
              }
              frame "Exit" {
                n652 = for {
                  shift-right: [w1876] -> w1873
                  shift-left: w1870 -> [w1877]
                  tunnel: string[] ["STOP", "RESET ENCODERS", "RESET YAW", "ARDUINO MODE 0"] -> [w1875] mode=indexing
                  n653 = Enqueue Element(queue=w1877, element=w1875) -> (queue out=w1876:refnum<queue>)  [unwired: 2 in, 2 out]
                }
              }
            }
          }
          frame 36 {
            # ">>> yStepper command>>>"
            # ">> Manual override >>"
            n654 = Dequeue Element(queue=w1888, timeout in ms (-1)=w1887, error in (no error)=w1886) -> (element=w1885:T10)  [unwired: 3 out]
            n655 = case shown="\"Start Task 1\", Default" w1885 {
              tunnel: [w1897 State_Type_Definitions,_for_0.26g_versions_and_later_2."True Stop" ("Enum")] -> w1890
              tunnel: [w1900 w1917] -> w1883
              tunnel: [State_Type_Definitions,_for_0.26g_versions_and_later_2."Idle" ("Enum") State_Type_Definitions,_for_0.26g_versions_and_later_2."Shutdown" ("Enum")] -> w1882
              tunnel: w1884 -> [w1891 _]
              tunnel: w1889 -> [w1896 w1914]
              tunnel: w1880 -> [w1895 _]
              frame "Start Task 1", Default {
                # ">> Is time up? >>"
                # "Determines if object is in range to pick up"
                # ">> Manual override >>"
                n656 = case shown="True" w1895 {
                  tunnel: [w1904 w1910] -> w1900
                  tunnel: w1896 -> [w1902 w1908]
                  frame False {
                    n657 = for {
                      tunnel: string[] ["CLOSE CLAW", "START TIMER"] ("element") -> [w1905] mode=indexing